vi "reconstruct 3D oblique image without config-2 (SubVI).vi"(0 "correction":T2={"vibration removal"=FALSE, "x correct fast/slow"=TRUE, "y correct fast/slow"=TRUE, "z correct fast/slow"=TRUE}, 1 "auto z adjust":T1={"margin"=100.0, "auto z adj"=FALSE, "average"=10, "use given ofst"=FALSE, "given ofst"=10}, 5 "image in":u16[][][](array[numeric])=array4x300x2304[2764800 elements], 7 "config in":T3={"xy cut pos correct"=[[0.0, 0.0, 0.0, 0.0], [0.0, 0.0, 0.0, 0.0], [0.0, 0.0, 0.0, 0.0], [0.0, 0.0, 0.0, 0.0], [0.0, 0.0, 0.0, 0.0], [0.0, 0.0, 0.0, 0.0], [0.0, 0.0, 0.0, 0.0], [0.0, 0.0, 0.0, 0.0], [0.0, 0.0, 0.0, 0.0], [0.0, 0.0, 0.0, 0.0], [0.0, 0.0, 0.0, 0.0], [0.0, 0.0, 0.0, 0.0], [0.0, 0.0, 0.0, 0.0], [0.0, 0.0, 0.0, 0.0], [0.0, 0.0, 0.0, 0.0], [0.0, 0.0, 0.0, 0.0], [0.0, 0.0, 0.0, 0.0], [0.0, 0.0, 0.0, 0.0], [0.0, 0.0, 0.0, 0.0], [0.0, 0.0, 0.0, 0.0], [0.0, 0.0, 0.0, 0.0], [0.0, 0.0, 0.0, 0.0], [0.0, 0.0, 0.0, 0.0], [0.0, 0.0, 0.0, 0.0]], "3D reconst config"={"xyz pos"=[46, 31, 52], "color 4"={"color array"=[0, 8388736, 16711680, 16776960, 16776960, 16711680, 16448250, 16448250], "num of colors"=4, "max"=7000.900000000023, "min"=100.0}, "autogain"=TRUE, "zoom"=1.0, "slice(T)/stack(F)"=FALSE, "xy cut mag"=0.9999999999999872, "xy cut ofst"=10.0, "z/xy comp"=0.9999999999999996, "y shift comp"=2.0, "max plot"=TRUE, "oblique angle [deg]"=45.0, "voxel size z [um]"=0.2909342537087903, "voxel size xy[um]"=0.20475, "reverse v"=FALSE, "reverse h"=TRUE, "3D reconstruction"=TRUE, "reverse z"=FALSE}, "xy cut pos"=[[0.0, 1.037506591193278, 0.966249270369417, 0.9158940969875857], [92.08631074928655, 92.74282819847565, 92.97750230838835, 92.67727146331777], [184.28758330950427, 185.01250778668418, 185.4134489785189, 184.69137479417213], [276.0489606758347, 276.53636075026884, 276.69217675847005, 276.4860055768869], [368.07921566607354, 368.89819980674065, 368.8136411193633, 368.38419699919905], [461.798744208641, 461.9849633403935, 462.2490904762467, 462.24814037863575], [554.7781467122519, 555.268397079519, 555.2332434679125, 554.7296917340917], [647.2882009960379, 647.5846314506646, 647.6995932615935, 647.5152743250628], [740.8889673372312, 741.2737568696792, 741.2034496464664, 740.8557139208467], [833.9643296995517, 834.1876026381326, 834.4726319214276, 834.3510194272217], [926.4886354475025, 926.7024074099736, 926.5560923778821, 926.5332900352184], [1019.2086613033152, 1019.556397028935, 1019.5734987859327, 1019.5449958576031], [1112.8274794991178, 1113.0498023400878, 1112.7296194451865, 1112.9329403339368], [1205.8866902020513, 1205.9931011344815, 1205.9531970348203, 1205.9037919590492], [1298.9126474886007, 1298.899346122047, 1299.058012423081, 1299.116918474962], [1392.299641867323, 1392.3689989929248, 1391.9509560440924, 1392.082069514408], [1485.6457820487744, 1485.6942370269344, 1485.3132478849304, 1485.3569523750357], [1578.3297041953701, 1578.9007128595708, 1578.61948396672, 1578.8503576861888], [1671.6273893986595, 1671.6549422293779, 1671.4050665576897, 1671.3604119699735], [1764.8661685500688, 1764.862368159625, 1764.8129630838534, 1765.1844512497485], [1857.8854751533427, 1857.8854751533427, 1857.6869047526473, 1857.7192080714206], [1951.1917112351302, 1951.1964617231852, 1951.2800703129517, 1951.4168843689333], [2043.5326481441634, 2043.787274303907, 2043.6352586861497, 2043.5982048793212], [2136.2422229262547, 2136.4265418627856, 2136.2099196074814, 2136.124410822493]], "AOD scan speed ratio"=5.0, "Nx"=93.5, "stack method"=enum."0pad to x and rot", "y shift"=3}, 9 "cropcalib":bool, 11 "cropcalib data":dbl[][][](array[numeric])=[[[330.8512624722854, 1176.151016996622, 0.0, 0.009428316830650669], [328.5787621076082, 1180.3546677235079, 0.0, 0.009179659527843352], [329.1155115826025, 1185.5118549945614, 0.0, 0.008879926465064643], [328.4474666338575, 1190.066406913501, 0.0, 0.00862012495571322]], [[327.58384877552515, 1179.3399452115818, 0.0, 0.009239326761173557], [330.64586772559215, 1183.570509586454, 0.0, 0.008992065492687374], [329.1182426075196, 1188.7090456628334, 0.0, 0.008697068994156926], [331.0833292234464, 1193.2988555935556, 0.0, 0.008438543533451089]], [[328.7041098476068, 1182.569513173517, 0.0, 0.009050212846350443], [330.5655883182281, 1186.770481635967, 0.0, 0.008807670479919528], [328.3880581820918, 1191.9068661319957, 0.0, 0.00851645191863399], [330.8192081039448, 1196.484526211637, 0.0, 0.008261875826756079]], [[329.0291138405168, 1185.8638941976924, 0.0, 0.00885968095793796], [330.2239592659729, 1190.0021055331606, 0.0, 0.008623760711384792], [329.88360431477196, 1195.207928124911, 0.0, 0.00833239920230058], [329.0055546600167, 1200.7794531816844, 0.0, 0.008027295813293513]], [[330.24527413712724, 1189.0833512123208, 0.0, 0.008675809944263788], [328.9577860583197, 1193.1902259931223, 0.0, 0.0084446078534114], [328.4487732377894, 1198.4548030016394, 0.0, 0.008153748883619465], [330.0763524036554, 1204.0443558848656, 0.0, 0.00785175048715124]], [[327.9606329363599, 1192.2041314919686, 0.0, 0.008499777889598343], [330.446114732459, 1196.4188076408827, 0.0, 0.008265497412007088], [331.55926553798633, 1201.6905041902264, 0.0, 0.007978069360316281], [330.71140004975507, 1207.1845836973916, 0.0, 0.0076851779540676735]], [[329.5691345378466, 1195.4239688330229, 0.0, 0.008320438746162742], [330.7306447795087, 1200.618390032539, 0.0, 0.008036017910836857], [329.65318996509365, 1204.906703846507, 0.0, 0.007805785611196943], [330.4225359020906, 1210.364940978633, 0.0, 0.0075187501899264125]], [[328.35008836956763, 1198.6407415088522, 0.0, 0.008143589762204376], [328.90402303435104, 1203.8024115267247, 0.0, 0.007864676757548733], [328.8872850578613, 1208.09777539, 0.0, 0.007637156351356103], [328.3105695920642, 1213.5593257233536, 0.0, 0.007353896502053807]], [[328.6451967358637, 1127.9703327325547, 0.0, 0.012550072767244045], [328.19424909379455, 1133.085548853325, 0.0, 0.012195479564778025], [328.3679132256721, 1137.3419122345406, 0.0, 0.011904528149263727], [329.8664011804312, 1142.824068114119, 0.0, 0.011535328382056603]], [[329.0137931176627, 1131.1684730544375, 0.0, 0.012327745071188015], [329.43921945403974, 1136.330837065185, 0.0, 0.011973302642268695], [330.07216132208566, 1140.623130285924, 0.0, 0.01168279908476291], [328.1737251840431, 1145.9867948563115, 0.0, 0.0113251919030582]], [[330.1899355869486, 1134.39359452557, 0.0, 0.012105667313626528], [328.70790882861525, 1139.5021004338992, 0.0, 0.011758300895061025], [328.0782246591683, 1143.8377820926603, 0.0, 0.01146774697568997], [329.54950432096183, 1149.2241857413321, 0.0, 0.011112275930991233]], [[331.42214147724894, 1137.5528595644162, 0.0, 0.011890206002647927], [330.97763687982894, 1142.7297019826956, 0.0, 0.01154163045813605], [330.54961412343954, 1147.0781334797975, 0.0, 0.011253169866028413], [327.0844397044803, 1152.4396225757132, 0.0, 0.010902999394719153]], [[330.929575643222, 1140.7785447879169, 0.0, 0.011672352543176941], [328.8439266492678, 1145.8708900077258, 0.0, 0.011332855690938066], [331.16506613573154, 1151.328789104024, 0.0, 0.010975049855985547], [332.3144635692056, 1155.6809834714056, 0.0, 0.010694261336075706]], [[328.87791169340977, 1143.9447348598565, 0.0, 0.011460629308520941], [328.60841680034633, 1149.0313226737098, 0.0, 0.011124898082049313], [328.28437086297305, 1154.4927373292637, 0.0, 0.010770522200949609], [327.16287039111825, 1158.8764418635192, 0.0, 0.010490677347170251]], [[329.35729265333816, 1147.090501489575, 0.0, 0.011252355087675737], [328.14957842477327, 1152.2634326180323, 0.0, 0.010914409859878342], [328.4917513371784, 1157.727572410442, 0.0, 0.01056362038447542], [330.95966686347083, 1162.1495563864858, 0.0, 0.01028441907635147]], [[329.1515568019215, 1151.3685299195897, 0.0, 0.010972467680426496], [332.2082161856812, 1155.482901454856, 0.0, 0.010706953165264467], [329.86557476312265, 1160.9761057095386, 0.0, 0.010358099929698581], [326.6180198128402, 1165.2756124065388, 0.0, 0.010089585308586238]], [[328.2018949478854, 1154.6071079334506, 0.0, 0.010763168859236505], [326.6757431393615, 1158.6721466023419, 0.0, 0.010503627582312526], [329.0019237207534, 1164.24453850444, 0.0, 0.010153614215199027], [330.29906981784274, 1168.5264642776929, 0.0, 0.009889219147039267]], [[330.7756952264671, 1157.893428641218, 0.0, 0.010553072495697563], [331.7656713031102, 1161.921777606122, 0.0, 0.010298698065293217], [328.3819521167621, 1167.4401073598385, 0.0, 0.00995592141258132], [329.42308717648444, 1171.686971815366, 0.0, 0.009696625521530881]], [[330.0486596989607, 1161.1143527630184, 0.0, 0.0103494039902354], [329.1844277898541, 1165.0713046949666, 0.0, 0.01010225437575639], [328.8711921864445, 1170.6878812751677, 0.0, 0.009757272221675928], [330.1502018730359, 1175.9537054449938, 0.0, 0.009440083845015646]], [[330.0279911009871, 1164.3021214095252, 0.0, 0.01015003229395419], [328.95127385724874, 1168.2935980154227, 0.0, 0.009903495516852285], [328.85226629139345, 1173.9565370919474, 0.0, 0.009559669235622265], [328.60848310183206, 1179.144742459143, 0.0, 0.009250831019732907]], [[329.797813873803, 1167.4416972495085, 0.0, 0.00995582360599151], [330.2854633911041, 1171.5422434795005, 0.0, 0.009705397308885887], [328.7652670570403, 1177.1705548368723, 0.0, 0.009367651211476397], [329.8191554231605, 1182.350456061726, 0.0, 0.009062967328391715]], [[328.76403530096667, 1170.631972332091, 0.0, 0.009760672437718717], [328.55523679710865, 1175.8083846400932, 0.0, 0.00944875576806857], [331.14545931703805, 1180.3934166639754, 0.0, 0.00917738553352469], [330.6972097456994, 1185.5925133499545, 0.0, 0.008875285435237572]], [[330.6527669048852, 1173.9082717155898, 0.0, 0.00956257006524093], [329.370737307894, 1179.0415869795693, 0.0, 0.009256913871127877], [330.81783725373816, 1183.6004158389724, 0.0, 0.008990331666880891], [328.0387873941186, 1188.7560952119093, 0.0, 0.008694395054772111]], [[327.27231388978987, 1177.0924704019544, 0.0, 0.0093722893955023], [329.7294177817484, 1182.2906875157555, 0.0, 0.009066449162680675], [328.797293940435, 1186.8506176880321, 0.0, 0.008803081896203244], [328.1656445749852, 1191.9915781247635, 0.0, 0.008511698293876373]]], 12 "array":i32[](array[numeric]), 13 "create 2D img":bool=TRUE) -> (2 "voxel number":i32[](array[numeric])=[65, 299, 203], 3 "image size":dbl[](array[numeric])=[65.0, 299.0, 203.0], 4 "z ofst":dbl, 6 "combined img2":u16[][](array[numeric]), 8 "xyz2":u16[][][](array[numeric]), 10 "voxel size [um]":dbl[](array[numeric])=[0.20475, 0.20475, 0.20475], 14 "combined img":u16[][](array[numeric]), 15 "xyz":u16[][][](array[numeric]))   [LabVIEW 2024] (continued)
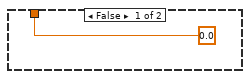
[diagram p3: hidden frame]
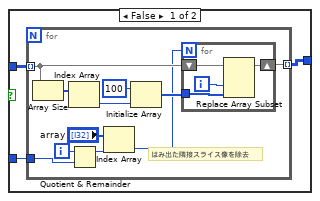
[diagram p4: hidden frame]
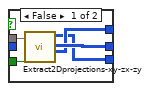
[diagram p6: hidden frame]
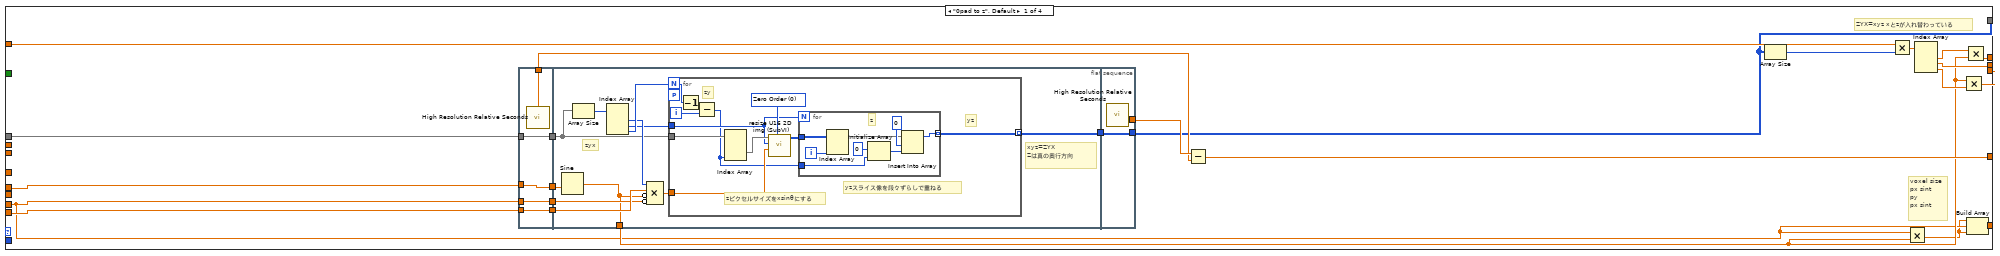
[diagram p7: hidden frame]
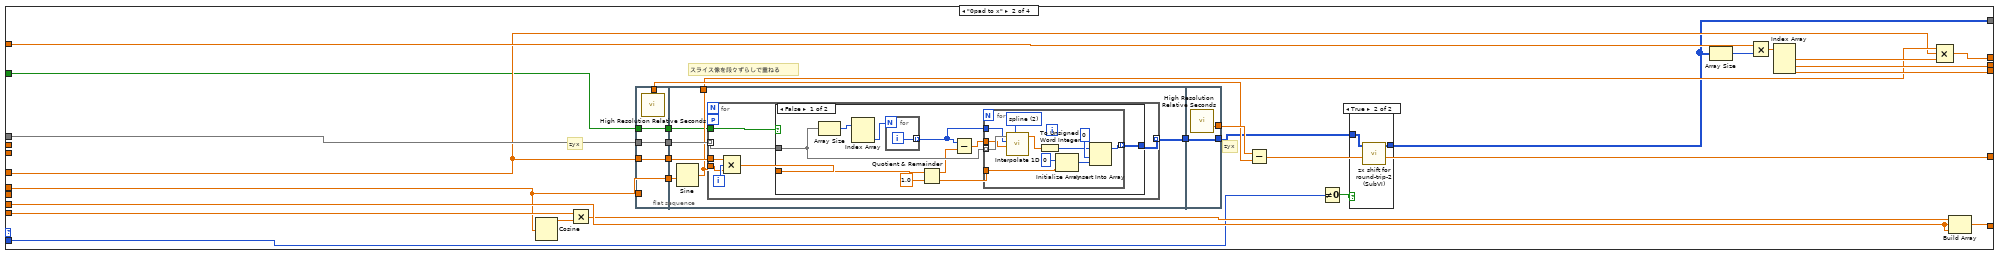
[diagram p8: hidden frame]
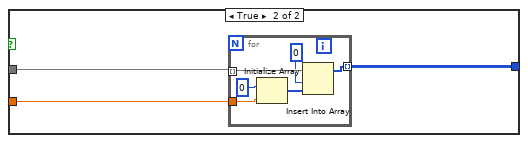
[diagram p10: hidden frame]
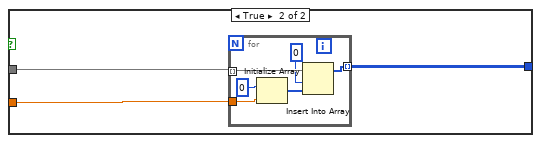
[diagram p12: hidden frame]
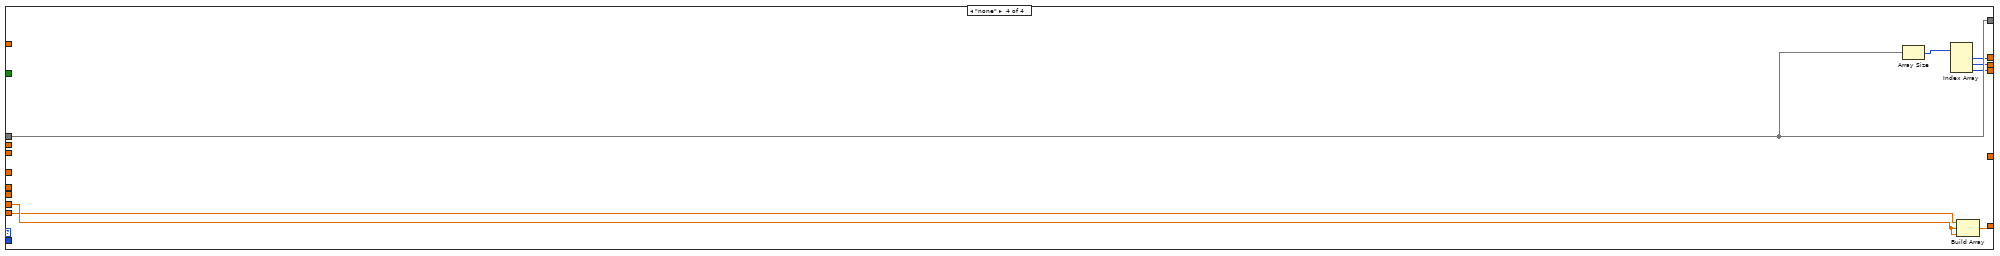
[diagram p13: hidden frame]
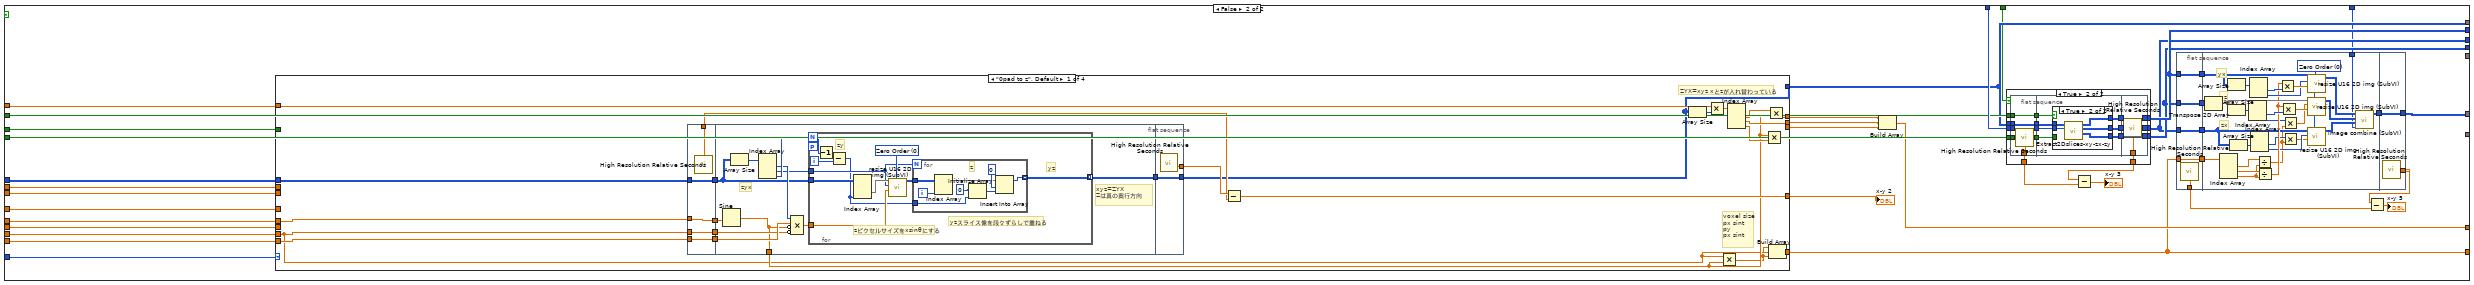
[diagram p14: hidden frame]
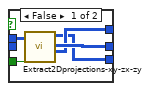
[diagram p16: hidden frame]
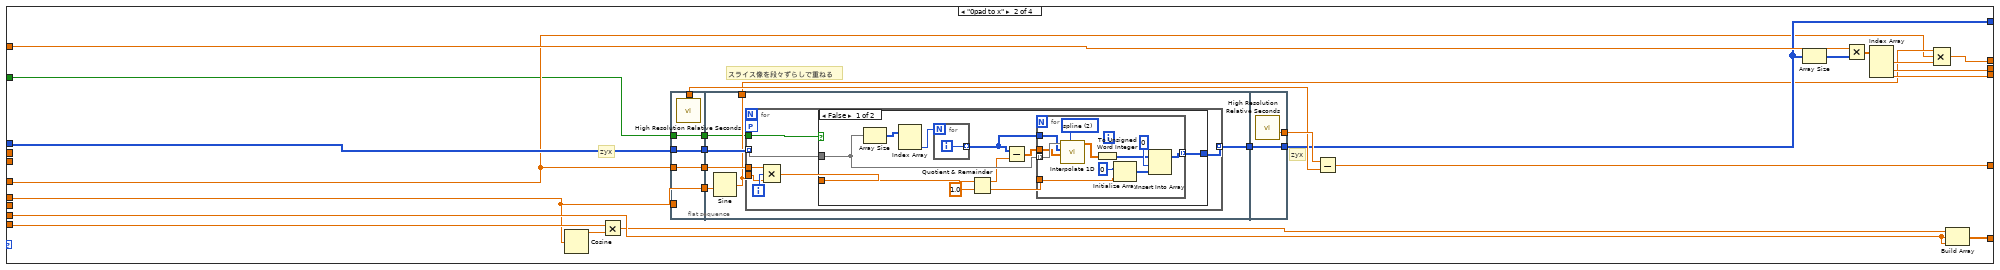
[diagram p17: hidden frame]
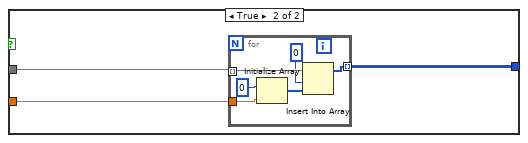
[diagram p18: hidden frame]
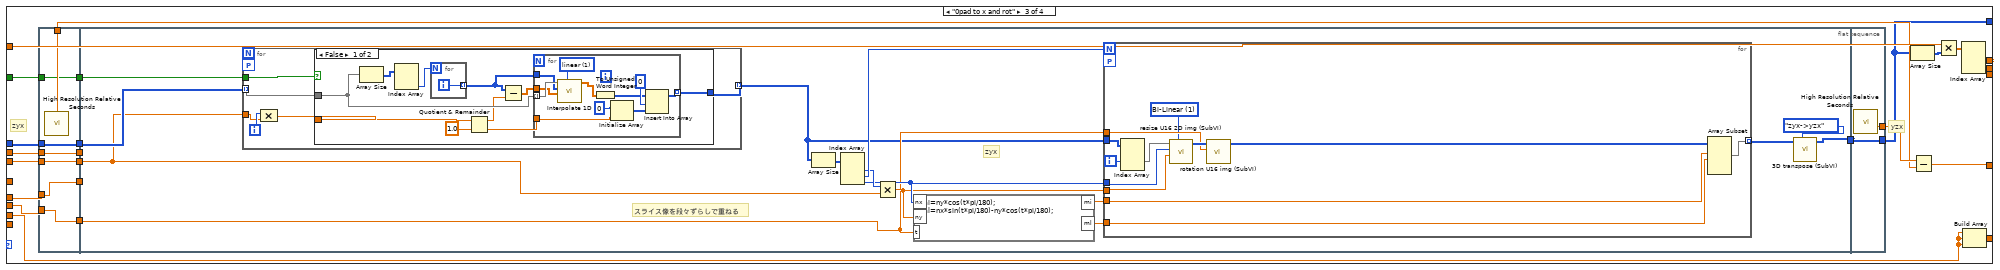
[diagram p19: hidden frame]
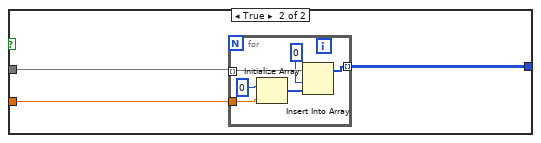
[diagram p20: hidden frame]
                            tunnel: w489 -> [w499] mode=indexing
                            tunnel: w490 -> [w502]
                            tunnel: [w500] -> w483 mode=indexing
                            tunnel: w485 -> [w498]
                            tunnel: w484 -> [w497]
                            w496 = 1 items=["nearest", "linear", "spline", "cubic Hermite", "Lagrange"] ("method")
                            n113 = call <vilib>:"Interpolate 1D.vi"("method"=w496, "xi"=w497, "X"=w498, "Y"=w499) -> ("yi"=w495:dbl[])  [unwired: 5 in, 2 out]
                            n114 = To Unsigned Word Integer(number=w495) -> (unsigned 16bit integer=w494:u16[])
                            n115 = Initialize Array(u16 0 ("element"), w502) -> (w501:u16[])
                            n116 = Insert Into Array(array=w494, index=0, new element=w501) -> (w500:u16[])
                          }
                        }
                        frame True {
                          n117 = for {
                            tunnel: w507 -> [w513] mode=indexing
                            tunnel: w506 -> [w510]
                            tunnel: [w508] -> w505 mode=indexing
                            n118 = Initialize Array(u16 0 ("element"), w510) -> (w509:u16[])
                            n119 = Insert Into Array(array=w513, index=0, new element=w509) -> (w508:u16[])
                          }
                        }
                      }
                    }
                    n120 = Not Equal To 0?(x=w458) -> (x != 0?=w457:bool)
                    n121 = case shown="True" w457 {
                      tunnel: w460 -> [w474 w476]
                      tunnel: [w474 w475] -> w459
                      frame False {
                      }
                      frame True {
                        n122 = call "zx shift for round-trip-2 (SubVI).vi"("input"=w476) -> ("output"=w475:u16[][][])  [unwired: 10 in]
                      }
                    }
                    n123 = Array Size(array=w459) -> (size(s)=w473:i32[])
                    n124 = Index Array(array=w473) -> (element #1=w471:i32, element #2=w472:i32, element #3=w470:i32)  [unwired: 3 in]
                    n125 = Multiply(x=w471, y=w462) -> (x*y=w469:dbl)
                    n126 = formula code="mi=ny*cos(t*pi/180);\nml=nx*sin(t*pi/180)-ny*cos(t*pi/180);"("nx"=w470, "ny"=w469, "t"=w464) -> ("mi"=w468:dbl, "ml"=w467:dbl)
                    n127 = for {
                      N: w472 -> [_]
                      tunnel: w459 -> [w525]
                      tunnel: w469 -> [w522]
                      tunnel: w470 -> [w521]
                      tunnel: [w514] -> w466 mode=indexing
                      tunnel: w464 -> [w519]
                      tunnel: w468 -> [w517]
                      tunnel: w467 -> [w516]
                      workers-P: _ -> [_]
                      i -> [w524]
                      w518 = u32 1 items=["Zero Order", "Bi-Linear", "Quadratic", "Cubic Spline"] ("Interpolation Type")
                      n128 = Index Array(array=w525, index (dim 1)=w524) -> (element=w523:u16[][])  [unwired: 2 in]
                      n129 = call "resize U16 2D img (SubVI).vi"("Interpolation Type"=w518, "Y Resolution"=w522, "X Resolution"=w521, "Array"=w523) -> ("Image Pixels (U16)"=w520:u16[][])  [unwired: 7 in]
                      n130 = call "rotation U16 img (SubVI).vi"("oblique angle [deg]"=w519, "Image Pixels (U16) in"=w520) -> ("Image Pixels (U16) out"=w515:u16[][])  [unwired: 9 in]
                      n131 = Array Subset(array=w515, index (row)=w517, length (row)=w516) -> (w514:u16[][])  [unwired: 2 in]
                    }
                    n132 = call "3D transpose (SubVI).vi"("Enum"=T6."zyx->yzx", "3D in"=w466) -> ("3D out"=w454:u16[][][])  [unwired: 9 in]
                    n133 = global read "global for picoscope.vi" "z cut length bottom"() -> (w452:u32)
                    n134 = Delete From Array(array=w454, length=w452) -> (array with subset deleted=w456:u16[][][])  [unwired: 3 in, 1 out]
                    n135 = global read "global for picoscope.vi" "z cut length top"() -> (w451:u32)
                    n136 = Delete From Array(array=w456, length=w451, index (dim 0)=0 ("index (page)")) -> (array with subset deleted=w453:u16[][][])  [unwired: 2 in, 1 out]
                  }
                  frame #2 {
                    n137 = call <vilib>:"High Resolution Relative Seconds.vi"() -> ("relative seconds"=w526:dbl)
                  }
                }
                n138 = Array Size(array=w425) -> (size(s)=w438:i32[])
                n139 = Subtract(x=w433, y=w432) -> (x-y=w431:dbl)
                n140 = Multiply(x=w434, y=w438) -> (x*y=w437:dbl[])
                n141 = Index Array(array=w437) -> (element #1=w424:dbl, element #2=w435:dbl, element #3=w436:dbl)  [unwired: 3 in]
                n142 = Build Array(w420, w420, w420) -> (w421:dbl[])
              }
              frame "none" {
                n143 = Array Size(array=w535) -> (size(s)=w529:i32[])
                n144 = Index Array(array=w529) -> (element #1=w534:i32, element #2=w533:i32, element #3=w532:i32)  [unwired: 3 in]
                n145 = Build Array(w528, w531, w531) -> (w530:dbl[])
              }
            }
            "x-y 9" <- w184
            n146 = Build Array(w176, w175, w174) -> (w173:dbl[])
            n147 = case shown="True" w163 {
              tunnel: w188 -> [_ w238]
              tunnel: w186 -> [_ w237]
              tunnel: w185 -> [_ w236]
              tunnel: [_ w235] -> w171
              tunnel: [_ w234] -> w170
              tunnel: w155 -> [_ w233]
              tunnel: [_ w232] -> w168
              tunnel: [_ w231] -> w167
              tunnel: [_ w230] -> w159
              frame False {
              }
              frame True {
                n148 = flat-sequence {
                  tunnel: w233 -> [w247]
                  tunnel: w236 -> [w248]
                  tunnel: w237 -> [w249]
                  tunnel: w238 -> [w250]
                  tunnel: [w250] -> w245
                  tunnel: [w249] -> w244
                  tunnel: [w248] -> w243
                  tunnel: [w247] -> w242
                  tunnel: [w246] -> w235
                  tunnel: [w254] -> w241
                  tunnel: [w253] -> w240
                  tunnel: [w252] -> w239
                  tunnel: w245 -> [w257]
                  tunnel: w244 -> [w256]
                  tunnel: w243 -> [w255]
                  tunnel: w242 -> [w251]
                  tunnel: [w269] -> w232
                  tunnel: [w270] -> w230
                  tunnel: [w271] -> w231
                  tunnel: w241 -> [w271]
                  tunnel: w240 -> [w270]
                  tunnel: w239 -> [w269]
                  tunnel: [w268] -> w234
                  frame #0 {
                    n149 = call <vilib>:"High Resolution Relative Seconds.vi"() -> ("relative seconds"=w246:dbl)
                  }
                  frame #1 {
                    n150 = case shown="True" w256 {
                      tunnel: [w260 w267] -> w252
                      tunnel: [w259 w266] -> w254
                      tunnel: [w261 w265] -> w253
                      tunnel: w251 -> [w262 w264]
                      tunnel: w257 -> [_ w263]
                      tunnel: w255 -> [w258 _]
                      frame False {
                        n151 = call "Extract2Dprojections-xy-zx-zy.vi"("max plot"=w258, "zyx"=w262) -> ("yx"=w260:u16[][], "zx"=w261:u16[][], "zy"=w259:u16[][])  [unwired: 7 in]
                      }
                      frame True {
                        n152 = call "Extract2Dslices-xy-zx-zy.vi"("xyz pos"=w263, "zyx"=w264) -> ("zy"=w266:u16[][], "zx"=w265:u16[][], "yx"=w267:u16[][])  [unwired: 7 in]
                      }
                    }
                  }
                  frame #2 {
                    n153 = call <vilib>:"High Resolution Relative Seconds.vi"() -> ("relative seconds"=w268:dbl)
                  }
                }
              }
            }
            n154 = Subtract(x=w170, y=w171) -> (x-y=→"x-y 8":dbl)
            n155 = flat-sequence {
              tunnel: w159 -> [w195]
              tunnel: w166 -> [w196]
              tunnel: w167 -> [w197]
              tunnel: w168 -> [w198]
              tunnel: [w198] -> w193
              tunnel: [w197] -> w192
              tunnel: [w196] -> w191
              tunnel: [w195] -> w190
              tunnel: [w194] -> w161
              tunnel: [w212] -> w189
              tunnel: w193 -> [w215]
              tunnel: w192 -> [w214]
              tunnel: w191 -> [w213]
              tunnel: w190 -> [w209]
              tunnel: w157 -> [w199]
              tunnel: [w229] -> w165
              tunnel: w189 -> [w229]
              tunnel: [w228] -> w162
              frame #0 {
                n156 = call <vilib>:"High Resolution Relative Seconds.vi"() -> ("relative seconds"=w194:dbl)
              }
              frame #1 {
                w200 = u32 0 items=["Zero Order", "Bi-Linear", "Quadratic", "Cubic Spline"] ("Interpolation Type")
                # "zx"
                # "yz"
                # "yx"
                n157 = Transpose 2D Array(2D array=w214) -> (transposed array=w220:u16[][])
                n158 = Index Array(array=w213) -> (element #1=w207:dbl, element #2=w217:dbl, element #3=w208:dbl)  [unwired: 3 in]
                n159 = Array Size(array=w220) -> (size(s)=w221:i32[])
                n160 = Array Size(array=w215) -> (size(s)=w227:i32[])
                n161 = Array Size(array=w209) -> (size(s)=w210:i32[])
                n162 = Index Array(array=w221) -> (element #1=w222:i32, element #2=w202:i32)  [unwired: 2 in]
                n163 = Index Array(array=w227) -> (element #1=w226:i32, element #2=w224:i32)  [unwired: 2 in]
                n164 = Index Array(array=w210) -> (element #1=w206:i32, element #2=w205:i32)  [unwired: 2 in]
                n165 = Divide(x=w207, y=w208) -> (x/y=w203:dbl)
                n166 = Divide(x=w217, y=w208) -> (x/y=w216:dbl)
                n167 = Multiply(x=w216, y=w226) -> (x*y=w225:dbl)
                n168 = Multiply(x=w216, y=w222) -> (x*y=w219:dbl)
                n169 = Multiply(x=w202, y=w203) -> (x*y=w201:dbl)
                n170 = Multiply(x=w206, y=w203) -> (x*y=w204:dbl)
                n171 = call "resize U16 2D img (SubVI).vi"("Interpolation Type"=w200, "Y Resolution"=w219, "X Resolution"=w201, "Array"=w220) -> ("Image Pixels (U16)"=w218:u16[][])  [unwired: 7 in]
                n172 = call "resize U16 2D img (SubVI).vi"("Interpolation Type"=w200, "Y Resolution"=w204, "X Resolution"=w205, "Array"=w209) -> ("Image Pixels (U16)"=w211:u16[][])  [unwired: 7 in]
                n173 = call "resize U16 2D img (SubVI).vi"("Interpolation Type"=w200, "Y Resolution"=w225, "X Resolution"=w224, "Array"=w215) -> ("Image Pixels (U16)"=w223:u16[][])  [unwired: 7 in]
                n174 = call "image combine (SubVI).vi"("spacing"=w199, "zx"=w211, "yz"=w218, "yx"=w223) -> ("combined"=w212:u16[][])  [unwired: 7 in]
              }
              frame #2 {
                n175 = call <vilib>:"High Resolution Relative Seconds.vi"() -> ("relative seconds"=w228:dbl)
              }
            }
            n176 = Subtract(x=w162, y=w161) -> (x-y=→"x-y 7":dbl)
          }
          n177 = Index Array(array=w142) -> (element #1=w126:u16[][][], element #2=w125:u16[][][])  [unwired: 8 in]
          n178 = Index Array(array=w123) -> (element #1=w122:u16[][], element #2=w121:u16[][])  [unwired: 6 in]
        }
        frame False {
          n179 = case shown="\"0pad to z\", Default" w547 {
            tunnel: w549 -> [w668 w735 w811 w895]
            tunnel: w559 -> [_ w718 _ _]
            tunnel: [w657 w723 w796 w894] -> w556
            tunnel: [w658 w731 w808 w892] -> w554
            tunnel: [w666 w730 w807 w893] -> w555
            tunnel: w567 -> [w669 w729 w806 _]
            tunnel: [w664 w726 w797 w895] -> w548
            tunnel: [w663 w725 w803 _] -> w564
            tunnel: w563 -> [w661 w717 w801 _]
            tunnel: w562 -> [w654 w720 w792 w891]
            tunnel: w561 -> [w655 w721 _ w888]
            tunnel: w560 -> [_ _ w799 _]
            tunnel: w558 -> [_ _ w798 _]
            tunnel: w557 -> [_ _ w794 _]
            tunnel: [w652 w719 w793 w890] -> w544
            tunnel: w542 -> [_ w714 w790 _]
            frame "0pad to z", Default {
              # "voxel size\npx sint\npy\npx sint"
              # "ZYX=xyz xとzが入れ替わっている"
              n180 = flat-sequence {
                tunnel: w668 -> [w680]
                tunnel: [w680] -> w675
                tunnel: [w679] -> w670
                tunnel: [w678] -> w662
                tunnel: w661 -> [w678]
                tunnel: [w677] -> w660
                tunnel: w654 -> [w677]
                tunnel: [w676] -> w659
                tunnel: w655 -> [w676]
                tunnel: w675 -> [w683]
                tunnel: [w681] -> w674
                tunnel: w662 -> [w690]
                tunnel: w660 -> [w688]
                tunnel: w659 -> [w689]
                tunnel: [w682] -> w656
                tunnel: [w712] -> w664
                tunnel: w674 -> [w712]
                tunnel: [w711] -> w671
                frame #0 {
                  n181 = call <vilib>:"High Resolution Relative Seconds.vi"() -> ("relative seconds"=w679:dbl)
                }
                frame #1 {
                  # "xyz=ZYX\nZは真の奥行方向"
                  # "zyx"
                  n182 = Sine(x=w690) -> (sin(x)=w682:dbl)
                  n183 = Array Size(array=w683) -> (size(s)=w691:i32[])
                  n184 = Index Array(array=w691) -> (element #1=w685:i32, element #2=w684:i32, element #3=w686:i32)  [unwired: 3 in]
                  n185 = Compound Arithmetic op=MULTIPLY(w685, w689, invert w682, invert w688) -> (w687:dbl)
                  n186 = for {
                    N: w686 -> [w695]
                    tunnel: w683 -> [w702]
                    tunnel: [w696] -> w681 mode=indexing
                    workers-P: _ -> [_]
                    tunnel: w684 -> [w697]
                    tunnel: w687 -> [w698]
                    i -> [w693]
                    w699 = u32 0 items=["Zero Order", "Bi-Linear", "Quadratic", "Cubic Spline"] ("Interpolation Type")
                    # "yz"
                    # "zピクセルサイズをxsinθにする"
                    # "yzスライス像を段々ずらしで重ねる"
                    # "zy"
                    n187 = Decrement(x=w695) -> (x-1=w694:i32)
                    n188 = Subtract(x=w694, y=w693) -> (x-y=w692:i32)
                    n189 = Index Array(array=w702, index (dim 2)=w692) -> (element=w701:u16[][])  [unwired: 2 in]
                    n190 = call "resize U16 2D img (SubVI).vi"("Interpolation Type"=w699, "Y Resolution"=w698, "X Resolution"=w697, "Array"=w701) -> ("Image Pixels (U16)"=w700:u16[][])  [unwired: 7 in]
                    n191 = for {
                      N: w697 -> [_]
                      tunnel: w700 -> [w710]
                      tunnel: [w706] -> w696 mode=indexing
                      tunnel: w692 -> [w705]
                      i -> [w703]
                      # "z"
                      n192 = Index Array(array=w710, index (col)=w703) -> (element=w704:u16[])  [unwired: 1 in]
                      n193 = Initialize Array(u16 0 ("element"), w705) -> (w707:u16[])
                      n194 = Insert Into Array(array=w704, index=0, new element=w707) -> (w706:u16[])
                    }
                  }
                }
                frame #2 {
                  n195 = call <vilib>:"High Resolution Relative Seconds.vi"() -> ("relative seconds"=w711:dbl)
                }
              }
              n196 = Subtract(x=w671, y=w670) -> (x-y=w663:dbl)
              n197 = Array Size(array=w664) -> (size(s)=w673:i32[])
              n198 = Multiply(x=w669, y=w673) -> (x*y=w672:dbl[])
              n199 = Multiply(x=w654, y=w656) -> (x*y=w653:dbl)
              n200 = Index Array(array=w672) -> (element #1=w667:dbl, element #2=w666:dbl, element #3=w665:dbl)  [unwired: 3 in]
              n201 = Multiply(x=w656, y=w665) -> (x*y=w658:dbl)
              n202 = Multiply(x=w667, y=w656) -> (x*y=w657:dbl)
              n203 = Build Array(w653, w654, w653) -> (w652:dbl[])
            }
            frame "0pad to x" {
              # "スライス像を段々ずらしで重ねる"
              # "zyx"
              # "zyx"
              n204 = Cosine(x=w717) -> (cos(x)=w715:dbl)
              n205 = Multiply(x=w721, y=w715) -> (x*y=w716:dbl)
              n206 = flat-sequence {
                tunnel: w718 -> [w742]
                tunnel: w735 -> [w743]
                tunnel: [w743] -> w738
                tunnel: [w742] -> w737
                tunnel: [w741] -> w727
                tunnel: [w740] -> w724
                tunnel: w717 -> [w740]
                tunnel: w714 -> [w739]
                tunnel: [w739] -> w713
                tunnel: w738 -> [w749]
                tunnel: w737 -> [w747]
                tunnel: [w748] -> w736
                tunnel: w724 -> [w746]
                tunnel: [w745] -> w722
                tunnel: w713 -> [w744]
                tunnel: [w789] -> w726
                tunnel: w736 -> [w789]
                tunnel: [w788] -> w728
                frame #0 {
                  n207 = call <vilib>:"High Resolution Relative Seconds.vi"() -> ("relative seconds"=w741:dbl)
                }
                frame #1 {
                  n208 = Sine(x=w746) -> (sin(x)=w745:dbl)
                  n209 = for {
                    tunnel: w749 -> [w756] mode=indexing
                    tunnel: w747 -> [w754]
                    tunnel: [w753] -> w748 mode=indexing
                    tunnel: w745 -> [w752]
                    tunnel: w744 -> [w751]
                    workers-P: _ -> [_]
                    i -> [w755]
                    n210 = Compound Arithmetic op=MULTIPLY(w754, w755, w752) -> (w750:dbl)
                    n211 = case shown="False" w751 {
                      tunnel: w756 -> [w762 w781]
                      tunnel: w750 -> [w766 w780]
                      tunnel: [w763 w779] -> w753
                      frame False {
                        n212 = Array Size(array=w762) -> (size(s)=w761:i32[])
                        n213 = Index Array(array=w761) -> (element #2=w760:i32)  [unwired: 2 in, 1 out]
                        n214 = for {
                          N: w760 -> [_]
                          tunnel: [w767] -> w758 mode=indexing
                          i -> [w767]
                        }
                        n215 = Quotient & Remainder(x=w766, y=1.0) -> (x-y*floor(x/y)=w759:dbl, floor(x/y)=w764:dbl)
                        n216 = Subtract(x=w758, y=w759) -> (x-y=w757:dbl[])
                        n217 = for {
                          tunnel: w762 -> [w773] mode=indexing
                          tunnel: w764 -> [w776]
                          tunnel: [w774] -> w763 mode=indexing
                          tunnel: w758 -> [w772]
                          tunnel: w757 -> [w771]
                          w770 = 2 items=["nearest", "linear", "spline", "cubic Hermite", "Lagrange"] ("method")
                          n218 = call <vilib>:"Interpolate 1D.vi"("method"=w770, "xi"=w771, "X"=w772, "Y"=w773) -> ("yi"=w769:dbl[])  [unwired: 5 in, 2 out]
                          n219 = To Unsigned Word Integer(number=w769) -> (unsigned 16bit integer=w768:u16[])
                          n220 = Initialize Array(u16 0 ("element"), w776) -> (w775:u16[])
                          n221 = Insert Into Array(array=w768, index=0, new element=w775) -> (w774:u16[])
                        }
                      }
                      frame True {
                        n222 = for {
                          tunnel: w781 -> [w787] mode=indexing
                          tunnel: w780 -> [w784]
                          tunnel: [w782] -> w779 mode=indexing
                          n223 = Initialize Array(u16 0 ("element"), w784) -> (w783:u16[])
                          n224 = Insert Into Array(array=w787, index=0, new element=w783) -> (w782:u16[])
                        }
                      }
                    }
                  }
                }
                frame #2 {
                  n225 = call <vilib>:"High Resolution Relative Seconds.vi"() -> ("relative seconds"=w788:dbl)
                }
              }
              n226 = Subtract(x=w728, y=w727) -> (x-y=w725:dbl)
              n227 = Array Size(array=w726) -> (size(s)=w734:i32[])
              n228 = Multiply(x=w729, y=w734) -> (x*y=w733:dbl[])
              n229 = Index Array(array=w733) -> (element #1=w732:dbl, element #2=w730:dbl, element #3=w731:dbl)  [unwired: 3 in]
              n230 = Compound Arithmetic op=MULTIPLY(w722, w718, w732) -> (w723:dbl)
              n231 = Build Array(w716, w720, w720) -> (w719:dbl[])
            }
            frame "0pad to x and rot" {
              # "yzx"
              # "zyx"
              n232 = flat-sequence {
                tunnel: w798 -> [w820]
                tunnel: w811 -> [w821]
                tunnel: [w821] -> w814
                tunnel: [w820] -> w813
                tunnel: [w819] -> w804
                tunnel: [w818] -> w802
                tunnel: w801 -> [w818]
                tunnel: [w817] -> w800
                tunnel: w799 -> [w817]
                tunnel: [w816] -> w795
                tunnel: w794 -> [w816]
                tunnel: [w815] -> w791
                tunnel: w790 -> [w815]
                tunnel: w814 -> [w825]
                tunnel: w813 -> [w824]
                tunnel: [w828] -> w812
                tunnel: w802 -> [_]
                tunnel: w800 -> [_]
                tunnel: w795 -> [w826]
                tunnel: w791 -> [w822]
                tunnel: [w887] -> w797
                tunnel: w812 -> [w887]
                tunnel: [w886] -> w805
                frame #0 {
                  n233 = call <vilib>:"High Resolution Relative Seconds.vi"() -> ("relative seconds"=w819:dbl)
                }
                frame #1 {
                  # "zyx"
                  # "スライス像を段々ずらしで重ねる"
                  n234 = for {
                    tunnel: w825 -> [w842] mode=indexing
                    tunnel: [w839] -> w823 mode=indexing
                    tunnel: w824 -> [w838]
                    tunnel: w822 -> [w837]
                    workers-P: _ -> [_]
                    i -> [w841]
                    n235 = Compound Arithmetic op=MULTIPLY(w841, w838) -> (w840:dbl)
                    n236 = case shown="False" w837 {
                      tunnel: w842 -> [w849 w867]
                      tunnel: w840 -> [w852 w866]
                      tunnel: [w843 w865] -> w839
                      frame False {
                        n237 = Array Size(array=w849) -> (size(s)=w848:i32[])
                        n238 = Index Array(array=w848) -> (element #2=w847:i32)  [unwired: 2 in, 1 out]
                        n239 = for {
                          N: w847 -> [_]
                          tunnel: [w853] -> w845 mode=indexing
                          i -> [w853]
                        }
                        n240 = Quotient & Remainder(x=w852, y=1.0) -> (x-y*floor(x/y)=w846:dbl, floor(x/y)=w850:dbl)
                        n241 = Subtract(x=w845, y=w846) -> (x-y=w844:dbl[])
                        n242 = for {
                          tunnel: w849 -> [w859] mode=indexing
                          tunnel: w850 -> [w862]
                          tunnel: [w860] -> w843 mode=indexing
                          tunnel: w845 -> [w858]
                          tunnel: w844 -> [w857]
                          w856 = 1 items=["nearest", "linear", "spline", "cubic Hermite", "Lagrange"] ("method")
                          n243 = call <vilib>:"Interpolate 1D.vi"("method"=w856, "xi"=w857, "X"=w858, "Y"=w859) -> ("yi"=w855:dbl[])  [unwired: 5 in, 2 out]
                          n244 = To Unsigned Word Integer(number=w855) -> (unsigned 16bit integer=w854:u16[])
                          n245 = Initialize Array(u16 0 ("element"), w862) -> (w861:u16[])
                          n246 = Insert Into Array(array=w854, index=0, new element=w861) -> (w860:u16[])
                        }
                      }
                      frame True {
                        n247 = for {
                          tunnel: w867 -> [w873] mode=indexing
                          tunnel: w866 -> [w870]
                          tunnel: [w868] -> w865 mode=indexing
                          n248 = Initialize Array(u16 0 ("element"), w870) -> (w869:u16[])
                          n249 = Insert Into Array(array=w873, index=0, new element=w869) -> (w868:u16[])
                        }
                      }
                    }
                  }
                  n250 = Array Size(array=w823) -> (size(s)=w836:i32[])
                  n251 = Index Array(array=w836) -> (element #1=w834:i32, element #2=w835:i32, element #3=w833:i32)  [unwired: 3 in]
                  n252 = Multiply(x=w834, y=w824) -> (x*y=w832:dbl)
                  n253 = formula code="mi=ny*cos(t*pi/180);\nml=nx*sin(t*pi/180)-ny*cos(t*pi/180);"("nx"=w833, "ny"=w832, "t"=w826) -> ("mi"=w831:dbl, "ml"=w830:dbl)
                  n254 = for {
                    N: w835 -> [_]
                    tunnel: w823 -> [w885]
                    tunnel: w832 -> [w882]
                    tunnel: w833 -> [w881]
                    tunnel: [w874] -> w829 mode=indexing
                    tunnel: w826 -> [w879]
                    tunnel: w831 -> [w877]
                    tunnel: w830 -> [w876]
                    workers-P: _ -> [_]
                    i -> [w884]
                    w878 = u32 1 items=["Zero Order", "Bi-Linear", "Quadratic", "Cubic Spline"] ("Interpolation Type")
                    n255 = Index Array(array=w885, index (dim 1)=w884) -> (element=w883:u16[][])  [unwired: 2 in]
                    n256 = call "resize U16 2D img (SubVI).vi"("Interpolation Type"=w878, "Y Resolution"=w882, "X Resolution"=w881, "Array"=w883) -> ("Image Pixels (U16)"=w880:u16[][])  [unwired: 7 in]
                    n257 = call "rotation U16 img (SubVI).vi"("oblique angle [deg]"=w879, "Image Pixels (U16) in"=w880) -> ("Image Pixels (U16) out"=w875:u16[][])  [unwired: 9 in]
                    n258 = Array Subset(array=w875, index (row)=w877, length (row)=w876) -> (w874:u16[][])  [unwired: 2 in]
                  }
                  n259 = call "3D transpose (SubVI).vi"("Enum"=T6."zyx->yzx", "3D in"=w829) -> ("3D out"=w828:u16[][][])  [unwired: 9 in]
                }
                frame #2 {
                  n260 = call <vilib>:"High Resolution Relative Seconds.vi"() -> ("relative seconds"=w886:dbl)
                }
              }
              n261 = Array Size(array=w797) -> (size(s)=w810:i32[])
              n262 = Subtract(x=w805, y=w804) -> (x-y=w803:dbl)
              n263 = Multiply(x=w806, y=w810) -> (x*y=w809:dbl[])
              n264 = Index Array(array=w809) -> (element #1=w796:dbl, element #2=w807:dbl, element #3=w808:dbl)  [unwired: 3 in]
              n265 = Build Array(w792, w792, w792) -> (w793:dbl[])
            }
            frame "none" {
              n266 = Array Size(array=w895) -> (size(s)=w889:i32[])
              n267 = Index Array(array=w889) -> (element #1=w894:i32, element #2=w893:i32, element #3=w892:i32)  [unwired: 3 in]
              n268 = Build Array(w888, w891, w891) -> (w890:dbl[])
            }
          }
          "x-y 2" <- w564
          n269 = Build Array(w556, w555, w554) -> (w553:dbl[])
          n270 = case shown="True" w541 {
            tunnel: w568 -> [_ w618]
            tunnel: w566 -> [_ w617]
            tunnel: w565 -> [_ w616]
            tunnel: [_ w615] -> w551
            tunnel: [_ w614] -> w550
            tunnel: w548 -> [_ w613]
            tunnel: [_ w612] -> w546
            tunnel: [_ w611] -> w545
            tunnel: [_ w610] -> w537
            frame False {
            }
            frame True {
              n271 = flat-sequence {
                tunnel: w613 -> [w627]
                tunnel: w616 -> [w628]
                tunnel: w617 -> [w629]
                tunnel: w618 -> [w630]
                tunnel: [w630] -> w625
                tunnel: [w629] -> w624
                tunnel: [w628] -> w623
                tunnel: [w627] -> w622
                tunnel: [w626] -> w615
                tunnel: [w634] -> w621
                tunnel: [w633] -> w620
                tunnel: [w632] -> w619
                tunnel: w625 -> [w637]
                tunnel: w624 -> [w636]
                tunnel: w623 -> [w635]
                tunnel: w622 -> [w631]
                tunnel: [w649] -> w612
                tunnel: [w650] -> w610
                tunnel: [w651] -> w611
                tunnel: w621 -> [w651]
                tunnel: w620 -> [w650]
                tunnel: w619 -> [w649]
                tunnel: [w648] -> w614
                frame #0 {
                  n272 = call <vilib>:"High Resolution Relative Seconds.vi"() -> ("relative seconds"=w626:dbl)
                }
                frame #1 {
                  n273 = case shown="True" w636 {
                    tunnel: [w640 w647] -> w632
                    tunnel: [w639 w646] -> w634
                    tunnel: [w641 w645] -> w633
                    tunnel: w631 -> [w642 w644]
                    tunnel: w637 -> [_ w643]
                    tunnel: w635 -> [w638 _]
                    frame False {
                      n274 = call "Extract2Dprojections-xy-zx-zy.vi"("max plot"=w638, "zyx"=w642) -> ("yx"=w640:u16[][], "zx"=w641:u16[][], "zy"=w639:u16[][])  [unwired: 7 in]
                    }
                    frame True {
                      n275 = call "Extract2Dslices-xy-zx-zy.vi"("xyz pos"=w643, "zyx"=w644) -> ("zy"=w646:u16[][], "zx"=w645:u16[][], "yx"=w647:u16[][])  [unwired: 7 in]
                    }
                  }
                }
                frame #2 {
                  n276 = call <vilib>:"High Resolution Relative Seconds.vi"() -> ("relative seconds"=w648:dbl)
                }
              }
            }
          }
          n277 = Subtract(x=w550, y=w551) -> (x-y=→"x-y 3":dbl)
          n278 = flat-sequence {
            tunnel: w537 -> [w575]
            tunnel: w544 -> [w576]
            tunnel: w545 -> [w577]
            tunnel: w546 -> [w578]
            tunnel: [w578] -> w573
            tunnel: [w577] -> w572
            tunnel: [w576] -> w571
            tunnel: [w575] -> w570
            tunnel: [w574] -> w539
            tunnel: [w592] -> w569
            tunnel: w573 -> [w595]
            tunnel: w572 -> [w594]
            tunnel: w571 -> [w593]
            tunnel: w570 -> [w589]
            tunnel: w536 -> [w579]
            tunnel: [w609] -> w543
            tunnel: w569 -> [w609]
            tunnel: [w608] -> w540
            frame #0 {
              n279 = call <vilib>:"High Resolution Relative Seconds.vi"() -> ("relative seconds"=w574:dbl)
            }
            frame #1 {
              w580 = u32 0 items=["Zero Order", "Bi-Linear", "Quadratic", "Cubic Spline"] ("Interpolation Type")
              # "zx"
              # "yz"
              # "yx"
              n280 = Transpose 2D Array(2D array=w594) -> (transposed array=w600:u16[][])
              n281 = Index Array(array=w593) -> (element #1=w587:dbl, element #2=w597:dbl, element #3=w588:dbl)  [unwired: 3 in]
              n282 = Array Size(array=w600) -> (size(s)=w601:i32[])
              n283 = Array Size(array=w595) -> (size(s)=w607:i32[])
              n284 = Array Size(array=w589) -> (size(s)=w590:i32[])
              n285 = Index Array(array=w601) -> (element #1=w602:i32, element #2=w582:i32)  [unwired: 2 in]
              n286 = Index Array(array=w607) -> (element #1=w606:i32, element #2=w604:i32)  [unwired: 2 in]
              n287 = Index Array(array=w590) -> (element #1=w586:i32, element #2=w585:i32)  [unwired: 2 in]
              n288 = Divide(x=w587, y=w588) -> (x/y=w583:dbl)
              n289 = Divide(x=w597, y=w588) -> (x/y=w596:dbl)
              n290 = Multiply(x=w596, y=w606) -> (x*y=w605:dbl)
              n291 = Multiply(x=w596, y=w602) -> (x*y=w599:dbl)
              n292 = Multiply(x=w582, y=w583) -> (x*y=w581:dbl)
              n293 = Multiply(x=w586, y=w583) -> (x*y=w584:dbl)
              n294 = call "resize U16 2D img (SubVI).vi"("Interpolation Type"=w580, "Y Resolution"=w599, "X Resolution"=w581, "Array"=w600) -> ("Image Pixels (U16)"=w598:u16[][])  [unwired: 7 in]
              n295 = call "resize U16 2D img (SubVI).vi"("Interpolation Type"=w580, "Y Resolution"=w584, "X Resolution"=w585, "Array"=w589) -> ("Image Pixels (U16)"=w591:u16[][])  [unwired: 7 in]
              n296 = call "resize U16 2D img (SubVI).vi"("Interpolation Type"=w580, "Y Resolution"=w605, "X Resolution"=w604, "Array"=w595) -> ("Image Pixels (U16)"=w603:u16[][])  [unwired: 7 in]
              n297 = call "image combine (SubVI).vi"("spacing"=w579, "zx"=w591, "yz"=w598, "yx"=w603) -> ("combined"=w592:u16[][])  [unwired: 7 in]
            }
            frame #2 {
              n298 = call <vilib>:"High Resolution Relative Seconds.vi"() -> ("relative seconds"=w608:dbl)
            }
          }
          n299 = Subtract(x=w540, y=w539) -> (x-y=→"x-y 5":dbl)
        }
      }
      "image size" <- w60
      n300 = Array Size(array=w58) -> (size(s)=→"voxel number":i32[])
    }
  }
  "yx" <- w22
  "zx" <- w21
  "zy" <- w20
  "xyz" <- w19
  "voxel size [um]" <- w17
  "combined img" <- w8
  "z ofst" <- w4
  "xyz2" <- w2
  "combined img2" <- w1
  n301 = case shown="True" FALSE {
    tunnel: w19 -> [_ w922]
    frame False {
    }
    frame True {
      n302 = call "Extract2Dprojections-xy-zx-zy.vi"("max plot"=TRUE, "zyx"=w922) -> ("yx"=→"Intensity Graph 3":u16[][], "zx"=→"Intensity Graph 2":u16[][], "zy"=→"Intensity Graph":u16[][])  [unwired: 7 in]
    }
  }
